vi "UHR-Fleezers Control (host) - 10.0.vi"() -> ()   [LabVIEW 2009] (continued)
  n151 = call "IMAQ Create"("Image Name"="APD 2 Image", "Image Type"=w32) -> ("New Image"=w30:T2)  [unwired: 3 in, 1 out]
  n152 = call "IMAQ Create"("Image Name"="Det. X Image", "Image Type"=w32) -> ("New Image"=w29:T2)  [unwired: 3 in, 1 out]
  n153 = call "IMAQ Create"("Image Name"="Det. Y Image", "Image Type"=w32) -> ("New Image"=w28:T2)  [unwired: 3 in, 1 out]
  n154 = call-poly "VISA Configure Serial Port"("VISA resource name"="Harvard Syringe Pump Serial Port", "baud rate (9600)"=u32 115200, "stop bits (10: 1 bit)"=w25) -> ("VISA resource name out"=w22:refnum<visa-resource-name>, "error out"=w23:errorcluster)  [unwired: 4 in, 7 out]
  n155 = Bundle("New Image"=w31, "New Image"=w30, "New Image"=w29, "New Image"=w28) -> (w27:T21)  [unwired: 1 in]
  n156 = node-c288(i64 1 ("Period")) -> (w157:T22)  [unwired: 3 out]
  n157 = node-c288() -> (w52:T22)  [unwired: 4 out]
  n158 = node-c288() -> (w50:T22)  [unwired: 4 out]
  n159 = node-c288() -> (w54:T22)  [unwired: 4 out]
  n160 = node-c288() -> (w39:T22)  [unwired: 4 in]
  n161 = timed-loop "Acquire Data" {
    tunnel: w107 -> [w951]
    tunnel: w106 -> [w950]
    tunnel: [w984] -> w254
    tunnel: [w978] -> w252
    timing: w157 -> [_]
    timing-out: [_] -> w156
    tunnel: w27 -> [w773]
    stop <- "Stop All" stop-if-true
    w757 = "NI_ChannelName" ("name")
    n162 = node-c288() -> ()  [unwired: 2 out]
    n163 = case "Reset data stream" shown="True" "Reset" {
      tunnel: w951 -> [w3448 w3460]
      tunnel: w950 -> [w3447 w3459]
      tunnel: [w3448 w3457] -> w946
      tunnel: [w3447 w3456] -> w945
      frame #0 {
      }
      frame #1 {
        w3458 = TRUE ("AI to FIFO")
        w3464 = FALSE ("AI to FIFO")
        n164 = local write "Overflow (data lost)"(FALSE ("Overflow (data lost)")) -> ()
        n165 = xnode "Read/Write Control"("FPGA VI Reference In"=w3460, "error in"=w3459, "AI to FIFO"=w3464, "APD to FIFO"=w3464) -> ("FPGA VI Reference Out"=w3452:T20, "error out"=w3463:errorcluster)
        n166 = xnode "Invoke Method"("FPGA VI Reference In"=w3451, "error in"=w3463) -> ("FPGA VI Reference Out"=w3461:T20, "error out"=w3462:errorcluster)
        n167 = xnode "Invoke Method"("FPGA VI Reference In"=w3461, "error in"=w3462) -> ("FPGA VI Reference Out"=w3455:T20, "error out"=w3454:errorcluster)
        n168 = flat-sequence {
          tunnel: w3452 -> [w3469]
          tunnel: [w3469] -> w3451
          frame #0 {
            n169 = Wait (ms)(milliseconds to wait=u32 1000) -> ()  [unwired: 1 out]
          }
        }
        n170 = xnode "Invoke Method"("FPGA VI Reference In"=w3455, "error in"=w3454) -> ("FPGA VI Reference Out"=w3450:T20, "error out"=w3453:errorcluster)
        n171 = flat-sequence {
          tunnel: w3450 -> [w3467]
          tunnel: [w3467] -> w3449
          frame #0 {
            n172 = Wait (ms)(milliseconds to wait=u32 1000) -> ()  [unwired: 1 out]
          }
        }
        n173 = xnode "Read/Write Control"("FPGA VI Reference In"=w3449, "error in"=w3453, "AI to FIFO"=w3458, "APD to FIFO"=w3458) -> ("FPGA VI Reference Out"=w3457:T20, "error out"=w3456:errorcluster)
      }
    }
    n174 = Or(x="Start AOD Scan", y="Trap Raster Scan") -> (x .or. y?=w896:bool)
    n175 = And(x="Save scans", y=w896) -> (x .and. y?=w942:bool)
    n176 = case "Start AOM raster scan" shown="True" w896 {
      tunnel: w946 -> [w2584 w2594]
      tunnel: w945 -> [w2583 w2593]
      tunnel: [w2584 w2587] -> w944
      tunnel: [w2583 w2586] -> w943
      frame #0 {
      }
      frame #1 {
        n177 = case shown="True" "Restart DMA? (AOD)" {
          tunnel: [w2960 w2962] -> w2588
          tunnel: [w2959 w2961] -> w2589
          tunnel: w2594 -> [w2960 w2970]
          tunnel: w2593 -> [w2959 w2969]
          frame #0 {
          }
          frame #1 {
            w2966 = FALSE ("AI to FIFO")
            n178 = xnode "Read/Write Control"("FPGA VI Reference In"=w2970, "error in"=w2969, "AI to FIFO"=w2966, "APD to FIFO"=w2966) -> ("FPGA VI Reference Out"=w2968:T20, "error out"=w2967:errorcluster)
            n179 = xnode "Invoke Method"("FPGA VI Reference In"=w2968, "error in"=w2967) -> ("FPGA VI Reference Out"=w2972:T20, "error out"=w2971:errorcluster)
            n180 = local write "Overflow (data lost)"(FALSE ("Overflow (data lost)")) -> ()
            n181 = xnode "Invoke Method"("FPGA VI Reference In"=w2972, "error in"=w2971) -> ("FPGA VI Reference Out"=w2964:T20, "error out"=w2963:errorcluster)
            n182 = xnode "Invoke Method"("FPGA VI Reference In"=w2964, "error in"=w2963) -> ("FPGA VI Reference Out"=w2962:T20, "error out"=w2961:errorcluster)
          }
        }
        n183 = case shown="True" "Move MCL Also?" {
          tunnel: w2589 -> [w2597 w2703]
          tunnel: w2588 -> [w2598 w2704]
          tunnel: [w2596 w2707] -> w2587
          tunnel: [w2595 w2706] -> w2586
          frame #0 {
            w2599 = TRUE ("AI to FIFO")
            n184 = xnode "Read/Write Control"("FPGA VI Reference In"=w2598, "error in"=w2597, "AI to FIFO"=w2599, "APD to FIFO"=w2599, "Start scan"=w2599) -> ("FPGA VI Reference Out"=w2596:T20, "error out"=w2595:errorcluster)
          }
          frame #1 {
            w2700 = FALSE ("1D or 2D Scan?")
            w2705 = TRUE ("AI to FIFO")
            # "Count for MCL loop"
            # "N total cycles"
            # "N steps"
            # "V_int"
            n185 = local read "Scan Range (nm)"() -> (w2682:dbl)
            n186 = local read "Number of F/B Scans (AOD)"() -> (w2699:u16)
            n187 = Sign(1:w2682) -> (0:w2681:dbl)
            n188 = Compound Arithmetic op=MULTIPLY(w2682, "MCL Step Position Ratio", "MCL/AOM Scale Tweak") -> (w2686:dbl)
            n189 = Negate(x=w2681) -> (-x=w2678:dbl)
            n190 = Multiply(x=w2678, y="MCL Step Increment (V_int)") -> (x*y=w2680:dbl)
            n191 = Divide(x=w2686, y="MCL X Cal (nm/V)") -> (x/y=w2692:dbl)
            n192 = Multiply(x=32767.0 ("y"), y=w2692) -> (x*y=w2698:dbl)
            n193 = local read "Total Counts (ticks)"() -> (w2683:u32)
            n194 = local read "Cycles/step (AOD)"() -> (w2694:u64)
            n195 = local read "Scan steps (AOD)"() -> (w2695:u64)
            n196 = Divide(x=w2698, y=10.0) -> (x/y=w2691:dbl)
            n197 = Divide(x=w2691, y="MCL Step Increment (V_int)") -> (x/y=w2689:dbl)
            n198 = Absolute Value(x=w2689) -> (abs(x)=w2677:dbl)
            n199 = Compound Arithmetic op=MULTIPLY(w2695, w2694, w2683) -> (w2690:u64)
            n200 = local write "wait to reset values"(w2705) -> ()
            n201 = local write "MCL Scanning"(w2705) -> ()
            n202 = Divide(x=w2690, y=w2677) -> (x/y=w2687:dbl)
            "MCL Count" <- w2687
            n203 = xnode "Read/Write Control"("FPGA VI Reference In"=w2704, "error in"=w2703, "Scan steps (MCL)"=w2677, "Number of scans (MCL)"=w2699, "Cycles per step (MCL)"=u64 1, "Scan freq.  increment (MCL)"=w2680, "1D or 2D Scan?"=w2700, "MCL Scan Axis"=w2700, "Cont. Scan (MCL)"=w2700, "MCL count"=w2687) -> ("FPGA VI Reference Out"=w2702:T20, "error out"=w2701:errorcluster)
            n204 = xnode "Read/Write Control"("FPGA VI Reference In"=w2702, "error in"=w2701, "AI to FIFO"=w2705, "APD to FIFO"=w2705, "Start scan"=w2705, "Start scan (MCL)"=w2705) -> ("FPGA VI Reference Out"=w2707:T20, "error out"=w2706:errorcluster)
          }
        }
        n205 = local write "Trap Raster Scan"(FALSE ("Trap Raster Scan")) -> ()
        "Raster Scanning..." <- TRUE ("Scanning...")
      }
    }
    n206 = Compound Arithmetic op=OR("Start MCL Scan", "Confocal Image", "Confocal Linescan") -> (w894:bool)
    n207 = And(x="Save Data (MCL)", y=w894) -> (x .and. y?=w941:bool)
    n208 = case "Start MCL raster scan" shown="True" w894 {
      tunnel: w944 -> [w1743 w1758]
      tunnel: w943 -> [w1742 w1757]
      tunnel: [w1743 w1753] -> w771
      tunnel: [w1742 w1752] -> w770
      tunnel: [FALSE w1751] -> w927
      tunnel: "Start MCL Scan" -> [_ w1746]
      tunnel: "Confocal Image" -> [_ w1745]
      tunnel: "Confocal Linescan" -> [_ _]
      frame #0 {
      }
      frame #1 {
        w1751 = TRUE
        n209 = case shown="True" "Restart DMA? (MCL)" {
          tunnel: [w1995 w1997] -> w1756
          tunnel: [w1994 w1996] -> w1755
          tunnel: w1758 -> [w1995 w2005]
          tunnel: w1757 -> [w1994 w2004]
          frame #0 {
          }
          frame #1 {
            w2001 = FALSE ("AI to FIFO")
            n210 = xnode "Read/Write Control"("FPGA VI Reference In"=w2005, "error in"=w2004, "AI to FIFO"=w2001, "APD to FIFO"=w2001) -> ("FPGA VI Reference Out"=w2003:T20, "error out"=w2002:errorcluster)
            n211 = xnode "Invoke Method"("FPGA VI Reference In"=w2003, "error in"=w2002) -> ("FPGA VI Reference Out"=w2007:T20, "error out"=w2006:errorcluster)
            n212 = xnode "Invoke Method"("FPGA VI Reference In"=w2007, "error in"=w2006) -> ("FPGA VI Reference Out"=w1999:T20, "error out"=w1998:errorcluster)
            n213 = xnode "Invoke Method"("FPGA VI Reference In"=w1999, "error in"=w1998) -> ("FPGA VI Reference Out"=w1997:T20, "error out"=w1996:errorcluster)
            n214 = local write "Overflow (data lost)"(FALSE ("Overflow (data lost)")) -> ()
          }
        }
        n215 = case shown="False" w1746 {
          selector: w1746 -> [_ w1762]
          tunnel: w1745 -> [w1761 _]
          tunnel: [w1761 w1762] -> w1744
          frame #0 {
            n216 = property on="2D or 1D Scan" class="Bool (strict)"("Val(Sgnl)"=w1761) -> ()  [unwired: 2 in, 2 out]
            n217 = property on="Confocal Image" class="Bool (strict)"("Value"=FALSE ("Start Confocal Map")) -> ()  [unwired: 2 in, 2 out]
          }
          frame #1 {
          }
        }
        n218 = local write "MCL Scanning"(w1751) -> ()
        n219 = local read "AO1"() -> (w1748:dbl)
        n220 = local read "AO2"() -> (w1747:dbl)
        n221 = case shown="True" "Center Scan" {
          tunnel: w1756 -> [w1769 w1878]
          tunnel: w1755 -> [w1768 w1877]
          tunnel: [w1767 w1876] -> w1753
          tunnel: [w1766 w1875] -> w1752
          tunnel: [w1764 w1862] -> w1750
          tunnel: [w1763 w1861] -> w1749
          tunnel: w1748 -> [w1764 w1867]
          tunnel: w1747 -> [w1763 w1870]
          tunnel: w1744 -> [_ _]
          frame #0 {
            w1765 = TRUE ("AI to FIFO")
            n222 = xnode "Read/Write Control"("FPGA VI Reference In"=w1769, "error in"=w1768, "AI to FIFO"=w1765, "APD to FIFO"=w1765, "Start scan (MCL)"=w1765) -> ("FPGA VI Reference Out"=w1767:T20, "error out"=w1766:errorcluster)
          }
          frame #1 {
            w1874 = TRUE ("AI to FIFO")
            n223 = local read "Scan steps (MCL)"() -> (w1853:u64)
            n224 = local read "Scan lines (y)"() -> (w1849:u64)
            n225 = local read "Fast Scan Dir"() -> (w1860:bool)
            n226 = local read "Actual MCL Inc (V)"() -> (w1850:dbl)
            n227 = Decrement(x=w1849) -> (x-1=w1848:u64)
            n228 = Decrement(x=w1853) -> (x-1=w1852:u64)
            n229 = Multiply(x=w1850, y=w1848) -> (x*y=w1847:dbl)
            n230 = Divide(x=w1847, y=2.0) -> (x/y=w1857:dbl)
            n231 = Multiply(x=w1850, y=w1852) -> (x*y=w1851:dbl)
            n232 = Divide(x=w1851, y=2.0) -> (x/y=w1856:dbl)
            n233 = Select(t=w1856, s=w1860, f=w1857) -> (s? t:f=w1855:dbl)
            n234 = Select(t=w1857, s=w1860, f=w1856) -> (s? t:f=w1859:dbl)
            n235 = Subtract(x=w1867, y=w1859) -> (x-y=w1858:dbl)
            n236 = Subtract(x=w1870, y=w1855) -> (x-y=w1854:dbl)
            n237 = local read "2D or 1D Scan"() -> (w1872:bool)
            n238 = Not(x=w1860) -> (.not. x?=w1866:bool)
            n239 = Not(x=w1872) -> (.not. x?=w1868:bool)
            n240 = And(x=w1860, y=w1868) -> (x .and. y?=w1869:bool)
            n241 = And(x=w1868, y=w1866) -> (x .and. y?=w1871:bool)
            n242 = Select(t=w1870, s=w1871, f=w1854) -> (s? t:f=w1861:dbl)
            n243 = Select(t=w1867, s=w1869, f=w1858) -> (s? t:f=w1862:dbl)
            n244 = call "Volt to I16.vi"("Voltage In"=w1862) -> ("I16 Voltage Out"=w1865:i16)
            n245 = call "Volt to I16.vi"("Voltage In"=w1861) -> ("I16 Voltage Out"=w1864:i16)
            n246 = xnode "Read/Write Control"("FPGA VI Reference In"=w1878, "error in"=w1877, "AI to FIFO"=w1874, "APD to FIFO"=w1874, "Start scan (MCL)"=w1874, "AO1"=w1865, "AO2"=w1864) -> ("FPGA VI Reference Out"=w1876:T20, "error out"=w1875:errorcluster)
          }
        }
        "Initial Y" <- w1750
        "Initial X" <- w1749
        "wait to reset values" <- w1751
      }
    }
    n247 = local read "Trap Pos Elements/DMA read"() -> (w767:u32)
    n248 = local read "Trap AI Elements/DMA read"() -> (w855:u32)
    n249 = local read "APD Elements/DMA read"() -> (w812:u32)
    n250 = xnode "Get APD Data"("FPGA VI Reference In"=w771, "error in"=w770, "Number of Elements"=w812, "Timeout (ms)"=-1) -> ("Data"=w811:u32[], "Elements Remaining"=→"APD FIFO Elements Remaining":u32)  [unwired: 2 out]
    n251 = xnode "Invoke Method"("FPGA VI Reference In"=w771, "error in"=w770, "Number of Elements"=w767, "Timeout (ms)"=-1) -> ("Data"=w766:u64[], "Elements Remaining"=→"Trap Pos FIFO El Remaining":u32)  [unwired: 2 out]
    n252 = xnode "Get Trap Data"("FPGA VI Reference In"=w771, "error in"=w770, "Number of Elements"=w855, "Timeout (ms)"=-1 ("Timeout")) -> ("FPGA VI Reference Out"=w842:T20, "error out"=w841:errorcluster, "Data"=w964:u32[], "Elements Remaining"=w993:u32)
    "FIFO El. Rem." <- w993
    n253 = local read "Trap AI FIFO Depth"() -> (w995:u32)
    n254 = call "IR AOM word to freq - vec.vi"("Frequency Word In (double vec)"=w766) -> ("Frequency Out"=w765:dbl[])
    n255 = Subtract(x=w995, y=w855) -> (x-y=w994:u32)
    n256 = Divide(x=w993, y=w994) -> (x/y=w992:dbl)
    "Buffer Status" <- w992
    n257 = Decimate 1D Array(w765) -> (w764:dbl[], w763:dbl[])
    n258 = Equal?(x=w992, y=1.0) -> (x = y?=w990:bool)
    n259 = Build Array(w764, w763) -> (w762:dbl[][])
    n260 = case "Alert buffer overflow" shown="True" w990 {
      frame #0 {
      }
      frame #1 {
        n261 = call <vilib>:"Beep.vi"() -> ()  [unwired: 3 in, 9 out]
        "Overflow (data lost)" <- TRUE ("Overflow (data lost)")
      }
    }
    n262 = local read "FPGA Averaging"() -> (w854:bool)
    n263 = case "Special unpacking case if no averaging done by FPGA" shown="False" w854 {
      tunnel: w964 -> [w2181 w2207]
      tunnel: [w2152 w2182] -> w963
      frame #0 {
        n264 = Decimate 1D Array(w2181) -> (w2180:u32[], w2179:u32[], w2178:u32[], w2177:u32[])
        n265 = Split Number(x=w2180) -> (hi(x)=w2176:u16[], lo(x)=w2175:u16[])
        n266 = Split Number(x=w2179) -> (hi(x)=w2174:u16[], lo(x)=w2173:u16[])
        n267 = Split Number(x=w2178) -> (hi(x)=w2172:u16[], lo(x)=w2171:u16[])
        n268 = Split Number(x=w2177) -> (hi(x)=w2170:u16[], lo(x)=w2169:u16[])
        n269 = To Word Integer(number=w2176) -> (16bit integer=w2168:i16[])
        n270 = To Word Integer(number=w2175) -> (16bit integer=w2167:i16[])
        n271 = To Word Integer(number=w2174) -> (16bit integer=w2166:i16[])
        n272 = To Word Integer(number=w2173) -> (16bit integer=w2165:i16[])
        n273 = To Word Integer(number=w2172) -> (16bit integer=w2164:i16[])
        n274 = To Word Integer(number=w2171) -> (16bit integer=w2163:i16[])
        n275 = To Word Integer(number=w2170) -> (16bit integer=w2162:i16[])
        n276 = To Word Integer(number=w2169) -> (16bit integer=w2161:i16[])
        n277 = To Double Precision Float(number=w2168) -> (double precision float=w2160:dbl[])
        n278 = To Double Precision Float(number=w2167) -> (double precision float=w2159:dbl[])
        n279 = To Double Precision Float(number=w2166) -> (double precision float=w2158:dbl[])
        n280 = To Double Precision Float(number=w2165) -> (double precision float=w2157:dbl[])
        n281 = To Double Precision Float(number=w2164) -> (double precision float=w2156:dbl[])
        n282 = To Double Precision Float(number=w2163) -> (double precision float=w2155:dbl[])
        n283 = To Double Precision Float(number=w2162) -> (double precision float=w2154:dbl[])
        n284 = To Double Precision Float(number=w2161) -> (double precision float=w2153:dbl[])
        n285 = Interleave 1D Arrays(w2160, w2159, w2158, w2157, w2156, w2155, w2154, w2153) -> (w2152:dbl[])
      }
      frame #1 {
        n286 = Decimate 1D Array(w2207) -> (w2198:u32[], w2196:u32[], w2194:u32[], w2192:u32[], w2190:u32[], w2188:u32[], w2186:u32[], w2184:u32[])
        n287 = To Long Integer(number=w2198) -> (32bit integer=w2206:i32[])
        n288 = To Long Integer(number=w2196) -> (32bit integer=w2205:i32[])
        n289 = To Long Integer(number=w2194) -> (32bit integer=w2204:i32[])
        n290 = To Long Integer(number=w2192) -> (32bit integer=w2203:i32[])
        n291 = To Long Integer(number=w2190) -> (32bit integer=w2202:i32[])
        n292 = To Long Integer(number=w2188) -> (32bit integer=w2201:i32[])
        n293 = To Long Integer(number=w2186) -> (32bit integer=w2200:i32[])
        n294 = To Long Integer(number=w2184) -> (32bit integer=w2199:i32[])
        n295 = To Double Precision Float(number=w2206) -> (double precision float=w2197:dbl[])
        n296 = To Double Precision Float(number=w2205) -> (double precision float=w2195:dbl[])
        n297 = To Double Precision Float(number=w2204) -> (double precision float=w2193:dbl[])
        n298 = To Double Precision Float(number=w2203) -> (double precision float=w2191:dbl[])
        n299 = To Double Precision Float(number=w2202) -> (double precision float=w2189:dbl[])
        n300 = To Double Precision Float(number=w2201) -> (double precision float=w2187:dbl[])
        n301 = To Double Precision Float(number=w2200) -> (double precision float=w2185:dbl[])
        n302 = To Double Precision Float(number=w2199) -> (double precision float=w2183:dbl[])
        n303 = Interleave 1D Arrays(w2197, w2195, w2193, w2191, w2189, w2187, w2185, w2183) -> (w2182:dbl[])
      }
    }
    n304 = local read "FPGA Ave."() -> (w853:dbl)
    n305 = local read "Trap Sets"() -> (w852:i16)
    n306 = Divide(x=w963, y=w853) -> (x/y=w970:dbl[])
    n307 = case "Deinterlace trap data, average down PSD" shown="2" w852 {
      tunnel: w970 -> [w2225 w2290]
      tunnel: [w2222 w2287] -> w845
      tunnel: [w2225 w2289] -> w744
      tunnel: "Detector Type" -> [w2224 w2285]
      tunnel: [w2223 w2288] -> w844
      tunnel: [w2221 w2286] -> w962
      frame #0 {
        n308 = Divide(x=w2225, y=3276.7) -> (x/y=w2226:dbl[])
        n309 = Decimate 1D Array(w2226) -> (w2235:dbl[], w2234:dbl[], w2233:dbl[], w2232:dbl[], w2231:dbl[], w2230:dbl[], w2229:dbl[], w2228:dbl[])
        n310 = case shown="\"IR-QPD + PSD + FB-QPD position\"" w2224 {
          tunnel: w2235 -> [w2259 w2284]
          tunnel: w2234 -> [w2258 w2283]
          tunnel: w2233 -> [w2243 w2261]
          tunnel: w2232 -> [w2244 w2271]
          tunnel: w2231 -> [w2257 w2282]
          tunnel: w2230 -> [w2256 w2281]
          tunnel: w2229 -> [w2240 w2262]
          tunnel: w2228 -> [w2239 w2260]
          tunnel: [w2238 w2268] -> w2223
          tunnel: [w2237 w2267] -> w2222
          tunnel: [w2236 w2266] -> w2221
          frame #0 {
            w2236 = 0  # Channel pattern
            n311 = Divide(x=w2259, y=w2244) -> (x/y=w2246:dbl[])
            n312 = Divide(x=w2258, y=w2244) -> (x/y=w2245:dbl[])
            n313 = Divide(x=w2257, y=w2240) -> (x/y=w2242:dbl[])
            n314 = Divide(x=w2256, y=w2239) -> (x/y=w2241:dbl[])
            n315 = Build Array(w2246, w2245, w2244, w2243, w2242, w2241, w2240, w2239) -> (w2237:dbl[][])
            n316 = Bundle("T1 Y", "T1 X", "T1 Sum", "FB Sum", "PSD Y", "PSD X", "PSD Y Sum", "PSD X Sum") -> (w2255:T34)  [unwired: 1 out]
            n317 = Cluster To Array(cluster=w2255) -> (array=w2238:string[])
          }
          frame #1 {
            w2266 = 3  # Channel pattern
            n318 = Negate(x=w2262) -> (-x=w2263:dbl[])
            n319 = Divide(x=w2284, y=w2271) -> (x/y=w2273:dbl[])
            n320 = Divide(x=w2283, y=w2271) -> (x/y=w2272:dbl[])
            n321 = Divide(x=w2282, y=w2262) -> (x/y=w2270:dbl[])
            n322 = Divide(x=w2281, y=w2263) -> (x/y=w2269:dbl[])
            n323 = Build Array(w2273, w2272, w2271, w2260, w2261, w2270, w2269, w2262) -> (w2267:dbl[][])
            n324 = Bundle("T1 Y", "T1 X", "T1 Sum", "FB X", "FB Sum", "PSD Y", "PSD X", "PSD Y Sum") -> (w2280:T34)  [unwired: 1 out]
            n325 = Cluster To Array(cluster=w2280) -> (array=w2268:string[])
          }
        }
      }
      frame #1 {
        n326 = case shown="\"IR-QPD + PSD + FB-QPD X position\"" w2285 {
          tunnel: w2290 -> [w2351 w2418 w2488]
          tunnel: [w2331 w2403 w2475] -> w2289
          tunnel: [w2317 w2394 w2466] -> w2288
          tunnel: [w2316 w2354 w2433] -> w2287
          tunnel: [w2310 w2392 w2464] -> w2286
          frame #0 {
            w2310 = 1  # Channel pattern
            # "time average x2 the 4th signal and the 4 psd signals (detection laser)"
            # "deinterlace 3 signals from qpd"
            n327 = Decimate 1D Array(w2351) -> (w2350:dbl[], w2349:dbl[], w2315:dbl[], w2348:dbl[], w2338:dbl[], w2336:dbl[], w2335:dbl[], w2333:dbl[])
            n328 = Decimate 1D Array(w2315) -> (w2314:dbl[], w2313:dbl[])
            n329 = Decimate 1D Array(w2350) -> (w2347:dbl[], w2319:dbl[])
            n330 = Decimate 1D Array(w2349) -> (w2346:dbl[], w2344:dbl[])
            n331 = Decimate 1D Array(w2348) -> (w2345:dbl[], w2343:dbl[])
            n332 = call "downsample 1D array - double.vi"("Ave N"=2.0, "Array In"=w2338) -> ("Array Out"=w2337:dbl[])  [unwired: 1 out]
            n333 = call "downsample 1D array - double.vi"("Ave N"=2.0, "Array In"=w2336) -> ("Array Out"=w2318:dbl[])  [unwired: 1 out]
            n334 = call "downsample 1D array - double.vi"("Ave N"=2.0, "Array In"=w2335) -> ("Array Out"=w2334:dbl[])  [unwired: 1 out]
            n335 = call "downsample 1D array - double.vi"("Ave N"=2.0, "Array In"=w2333) -> ("Array Out"=w2332:dbl[])  [unwired: 1 out]
            n336 = Interleave 1D Arrays(w2347, w2346, w2345, w2319, w2344, w2343, w2314, w2313, w2337, w2318, w2334, w2332) -> (w2331:dbl[])
            n337 = Divide(x=w2331, y=3276.7) -> (x/y=w2330:dbl[])
            n338 = Decimate 1D Array(w2330) -> (w2329:dbl[], w2328:dbl[], w2327:dbl[], w2326:dbl[], w2325:dbl[], w2324:dbl[], w2312:dbl[], w2311:dbl[], w2323:dbl[], w2322:dbl[], w2321:dbl[], w2320:dbl[])
            n339 = Divide(x=w2329, y=w2327) -> (x/y=w2297:dbl[])
            n340 = Divide(x=w2328, y=w2327) -> (x/y=w2296:dbl[])
            n341 = Divide(x=w2326, y=w2324) -> (x/y=w2295:dbl[])
            n342 = Divide(x=w2325, y=w2324) -> (x/y=w2294:dbl[])
            n343 = Divide(x=w2323, y=w2321) -> (x/y=w2293:dbl[])
            n344 = Divide(x=w2322, y=w2320) -> (x/y=w2292:dbl[])
            n345 = Build Array(w2297, w2296, w2327, w2295, w2294, w2324, w2312, w2311, w2293, w2292, w2321, w2320) -> (w2316:dbl[][])
            n346 = Bundle("T1 Y", "T1 X", "T1 Sum", "T2 Y", "T2 X", "T2 Sum", "T1 FB Sum", "T2 FB Sum", "PSD Y", "PSD X", "PSD Y Sum", "PSD X Sum") -> (w2298:T35)  [unwired: 1 out]
            n347 = Cluster To Array(cluster=w2298) -> (array=w2317:string[])
          }
          frame #1 {
            w2392 = 2  # Channel pattern
            # "time average x2 the 3 psd signals (detection laser)"
            # "deinterlace 3 signals from qpds"
            n348 = Decimate 1D Array(w2418) -> (w2417:dbl[], w2416:dbl[], w2393:dbl[], w2415:dbl[], w2406:dbl[], w2405:dbl[], w2404:dbl[], w2380:dbl[])
            n349 = Decimate 1D Array(w2393) -> (w2375:dbl[], w2373:dbl[])
            n350 = Decimate 1D Array(w2417) -> (w2414:dbl[], w2395:dbl[])
            n351 = Decimate 1D Array(w2416) -> (w2413:dbl[], w2411:dbl[])
            n352 = Decimate 1D Array(w2415) -> (w2412:dbl[], w2410:dbl[])
            n353 = Decimate 1D Array(w2380) -> (w2376:dbl[], w2374:dbl[])
            n354 = call "downsample 1D array - double.vi"("Ave N"=2.0, "Array In"=w2406) -> ("Array Out"=w2379:dbl[])  [unwired: 1 out]
            n355 = call "downsample 1D array - double.vi"("Ave N"=2.0, "Array In"=w2405) -> ("Array Out"=w2378:dbl[])  [unwired: 1 out]
            n356 = call "downsample 1D array - double.vi"("Ave N"=2.0, "Array In"=w2404) -> ("Array Out"=w2377:dbl[])  [unwired: 1 out]
            n357 = Interleave 1D Arrays(w2414, w2413, w2412, w2395, w2411, w2410, w2376, w2375, w2374, w2373, w2379, w2378, w2377) -> (w2403:dbl[])
            n358 = Divide(x=w2403, y=3276.7) -> (x/y=w2402:dbl[])
            n359 = Decimate 1D Array(w2402) -> (w2401:dbl[], w2400:dbl[], w2399:dbl[], w2398:dbl[], w2397:dbl[], w2396:dbl[], w2365:dbl[], w2363:dbl[], w2362:dbl[], w2360:dbl[], w2359:dbl[], w2358:dbl[], w2355:dbl[])
            n360 = Negate(x=w2355) -> (-x=w2353:dbl[])
            n361 = Divide(x=w2359, y=w2355) -> (x/y=w2357:dbl[])
            n362 = Divide(x=w2358, y=w2353) -> (x/y=w2356:dbl[])
            n363 = Divide(x=w2401, y=w2399) -> (x/y=w2384:dbl[])
            n364 = Divide(x=w2400, y=w2399) -> (x/y=w2383:dbl[])
            n365 = Divide(x=w2398, y=w2396) -> (x/y=w2382:dbl[])
            n366 = Divide(x=w2397, y=w2396) -> (x/y=w2381:dbl[])
            n367 = Divide(x=w2365, y=w2363) -> (x/y=w2364:dbl[])
            n368 = Divide(x=w2362, y=w2360) -> (x/y=w2361:dbl[])
            n369 = Build Array(w2384, w2383, w2399, w2382, w2381, w2396, w2364, w2363, w2361, w2360, w2357, w2356, w2355) -> (w2354:dbl[][])
            n370 = Bundle("T1 Y", "T1 X", "T1 Sum", "T2 Y", "T2 X", "T2 Sum", "T1 FB X", "T1 FB Sum", "T2 FB X", "T2 FB Sum", "PSD Y", "PSD X", "PSD Y Sum") -> (w2385:T36)  [unwired: 1 out]
            n371 = Cluster To Array(cluster=w2385) -> (array=w2394:string[])
          }
          frame #2 {
            w2464 = 4  # Channel pattern
            # "time average x2 the 3 psd signals (detection laser)"
            # "deinterlace 3 signals from qpds"
            n372 = Decimate 1D Array(w2488) -> (w2487:dbl[], w2486:dbl[], w2465:dbl[], w2485:dbl[], w2431:dbl[], w2477:dbl[], w2476:dbl[], w2453:dbl[])
            n373 = Decimate 1D Array "Feedback Sum"(w2465) -> (w2449:dbl[], w2447:dbl[])
            n374 = Decimate 1D Array "QPD Y"(w2487) -> (w2484:dbl[], w2467:dbl[])
            n375 = Decimate 1D Array "QPD X"(w2486) -> (w2483:dbl[], w2481:dbl[])
            n376 = Decimate 1D Array "Feedback Y"(w2431) -> (w2430:dbl[], w2429:dbl[])
            n377 = Decimate 1D Array "QPD Sum"(w2485) -> (w2482:dbl[], w2480:dbl[])
            n378 = Decimate 1D Array "Feedback X"(w2453) -> (w2450:dbl[], w2448:dbl[])
            n379 = call "downsample 1D array - double.vi"("Ave N"=2.0, "Array In"=w2477) -> ("Array Out"=w2452:dbl[])  [unwired: 1 out]
            n380 = call "downsample 1D array - double.vi"("Ave N"=2.0, "Array In"=w2476) -> ("Array Out"=w2451:dbl[])  [unwired: 1 out]
            n381 = Interleave 1D Arrays(w2484, w2483, w2482, w2467, w2481, w2480, w2430, w2450, w2449, w2429, w2448, w2447, w2452, w2451) -> (w2475:dbl[])
            n382 = Divide(x=w2475, y=3276.7) -> (x/y=w2474:dbl[])
            n383 = Decimate 1D Array(w2474) -> (w2473:dbl[], w2472:dbl[], w2471:dbl[], w2470:dbl[], w2469:dbl[], w2468:dbl[], w2426:dbl[], w2440:dbl[], w2424:dbl[], w2425:dbl[], w2438:dbl[], w2422:dbl[], w2436:dbl[], w2434:dbl[])
            n384 = Negate(x=w2434) -> (-x=w2432:dbl[])
            n385 = Divide(x=w2436, y=w2432) -> (x/y=w2435:dbl[])
            n386 = Divide(x=w2425, y=w2422) -> (x/y=w2421:dbl[])
            n387 = Divide(x=w2426, y=w2424) -> (x/y=w2423:dbl[])
            n388 = Divide(x=w2473, y=w2471) -> (x/y=w2457:dbl[])
            n389 = Divide(x=w2472, y=w2471) -> (x/y=w2456:dbl[])
            n390 = Divide(x=w2470, y=w2468) -> (x/y=w2455:dbl[])
            n391 = Divide(x=w2469, y=w2468) -> (x/y=w2454:dbl[])
            n392 = Divide(x=w2440, y=w2424) -> (x/y=w2439:dbl[])
            n393 = Divide(x=w2438, y=w2422) -> (x/y=w2437:dbl[])
            n394 = Build Array(w2457, w2456, w2471, w2455, w2454, w2468, w2423, w2439, w2424, w2421, w2437, w2422, w2435, w2434) -> (w2433:dbl[][])
            n395 = Bundle("T1 Y", "T1 X", "T1 Sum", "T2 Y", "T2 X", "T2 Sum", "T1 FB Y", "T1 FB X", "T1 FB Sum", "T2 FB Y", "T2 FB X", "T2 FB Sum", "PSD X", "PSD Y Sum") -> (w2420:T37)  [unwired: 1 out]
            n396 = Cluster To Array(cluster=w2420) -> (array=w2466:string[])
          }
        }
      }
    }
    "AI labels" <- w844
    n397 = To Word Integer(number=w744) -> (16bit integer=w749:i16[])
    n398 = Decimate 1D Array(w811) -> (w840:u32[], w775:u32[])
    n399 = local read "DMA Update Period (s)"() -> (w856:dbl)
    n400 = Build Array(w840, w775) -> (w924:u32[][])
    n401 = local read "Data Period (s)"() -> (w825:dbl)
    n402 = Decimate 1D Array(w744) -> (w742:dbl[], w741:dbl[], w739:dbl[], w738:dbl[])  [unwired: 9 out]
    n403 = To Double Precision Float(number=w924) -> (double precision float=w925:dbl[][])
    n404 = local read "APD Integration Time (s)"() -> (w788:dbl)
    n405 = Divide(x=w742, y=w741) -> (x/y=w743:dbl[])
    n406 = Divide(x=w739, y=w738) -> (x/y=w740:dbl[])
    n407 = feedback #1(0.0) -> (w759:dbl)
    n408 = Add(x=w856, y=w759) -> (x+y=w966:dbl)
    n409 = To Time Stamp(1:w759) -> (0:w758:timestamp)
    n410 = Split 1D Array(array=w743, index="N El. to Ave.") -> (second subarray=w747:dbl[])  [unwired: 1 out]
    n411 = Split 1D Array(array=w740, index="N El. to Ave.") -> (second subarray=w746:dbl[])  [unwired: 1 out]
    n412 = local read "Trap X AI1 (DMA)"() -> (w745:T10)
    n413 = Multiply(x=w825, y="Trap Disp. Downsample") -> (x*y=w760:dbl)
    "Display Period (s)" <- w760
    n414 = for "Trap AI" {
      tunnel: [w2220] -> w958 mode=indexing
      tunnel: w758 -> [w2210]
      tunnel: "Trap Disp. Downsample" -> [w2218]
      tunnel: w845 -> [w2216] mode=indexing
      tunnel: w825 -> [w2215]
      tunnel: w844 -> [w2214] mode=indexing
      tunnel: w757 -> [w2213]
      tunnel: [w2212] -> w799 mode=indexing
      tunnel: w760 -> [w2211]
      workers-P: _ -> [_]
      n415 = Bundle By Name("Y"=w2216, "dt"=w2215) -> (w2217:waveform(dbl))  [unwired: 1 out]
      n416 = Set Waveform Attribute(5:w2214, 6:w2213, 7:w2217) -> (3:w2212:waveform(dbl))  [unwired: 1 in, 2 out]
      n417 = call "downsample 1D array - double.vi"("Ave N"=w2218, "Array In"=w2216) -> ("Array Out"=w2219:dbl[])  [unwired: 1 out]
      n418 = Bundle By Name(cluster=w2212, "t0"=w2210, "Y"=w2219, "dt"=w2211) -> (w2220:waveform(dbl))
    }
    n419 = call <vilib>:"Mean.vi"("X"=w746) -> ("mean"=w733:dbl)  [unwired: 1 out]
    n420 = call <vilib>:"Mean.vi"("X"=w747) -> ("mean"=w734:dbl)  [unwired: 1 out]
    n421 = Reciprocal(x=w760) -> (1/x=→"Trap Disp. Freq. (Hz)":dbl)
    n422 = local read "Data points/scans (MCL)"() -> (w936:dbl)
    n423 = To Fixed-Point(number=w733) -> (fixed-point=w731:fxp<+/-,16,1>)  [unwired: 1 in]
    n424 = To Fixed-Point(number=w734) -> (fixed-point=w732:fxp<+/-,16,1>)  [unwired: 1 in]
    n425 = Bundle("Trap 1 Pos.", "Trap 2 Pos.") -> (w756:cluster{string, string})  [unwired: 1 out]
    n426 = Bundle By Name(cluster=w745, "Set 1"=w732, "Set 2"=w731) -> (→"Trap X AI1 (DMA)":T10)
    n427 = Cluster To Array(cluster=w756) -> (array=w753:string[])
    n428 = for "Trap Position" {
      tunnel: w762 -> [w1007] mode=indexing
      tunnel: "Trap Disp. Downsample" -> [w1006]
      tunnel: w760 -> [w1004]
      tunnel: w758 -> [w1003]
      tunnel: w757 -> [w1001]
      tunnel: w753 -> [w1000] mode=indexing
      tunnel: [w999] -> w752 mode=indexing
      n429 = call "downsample 1D array - double.vi"("Ave N"=w1006, "Array In"=w1007) -> ("Array Out"=w1005:dbl[])  [unwired: 1 out]
      n430 = Bundle By Name("Y"=w1005, "dt"=w1004, "t0"=w1003) -> (w1002:waveform(dbl))  [unwired: 1 out]
      n431 = Set Waveform Attribute(5:w1000, 6:w1001, 7:w1002) -> (3:w999:waveform(dbl))  [unwired: 1 in, 2 out]
    }
    "Trap Positions" <- w752
    n432 = Bundle("APD 1", "APD 2") -> (w957:cluster{string, string})  [unwired: 1 out]
    n433 = Cluster To Array(cluster=w957) -> (array=w954:string[])
    n434 = for "APD" {
      tunnel: w925 -> [w2143] mode=indexing
      tunnel: w788 -> [w2151]
      tunnel: [w2147] -> w795 mode=indexing
      tunnel: "APD Disp. Scale" -> [w2148]
      tunnel: w757 -> [w2146]
      tunnel: w954 -> [w2145] mode=indexing
      tunnel: "APD Disp. Downsample" -> [w2141]
      tunnel: [w2144] -> w953
      workers-P: _ -> [_]
      tunnel: w758 -> [w2140]
      n435 = call "integrate 1D array interval - double.vi"("Ave N"=w2141, "Array In"=w2143) -> ("Array Out"=w2142:dbl[])  [unwired: 1 out]
      n436 = Multiply(x=w2151, y=w2141) -> (x*y=w2144:dbl)
      n437 = Divide(x=w2142, y=w2148) -> (x/y=w2149:dbl[])
      n438 = Bundle By Name("t0"=w2140, "Y"=w2149, "dt"=w2144) -> (w2150:waveform(dbl))  [unwired: 1 out]
      n439 = Set Waveform Attribute(5:w2145, 6:w2146, 7:w2150) -> (3:w2147:waveform(dbl))  [unwired: 1 in, 2 out]
    }
    "APD Display Period (s)" <- w953
    n440 = Reciprocal(x=w953) -> (1/x=→"APD Display Freq. (Hz)":dbl)
    n441 = Increment(x=w936) -> (x+1=w937:dbl)
    n442 = To Double Precision Float(number=w840) -> (double precision float=w839:dbl[])
    n443 = feedback #2(w937) -> (w940:dbl)
    n444 = Select(t=0, s=w927, f=w940) -> (s? t:f=w933:dbl)
    n445 = Array Size(array=w839) -> (size(s)=w939:i32)
    n446 = Add(x=w939, y=w933) -> (x+y=w934:dbl)
    n447 = feedback #3(w840) -> (w923:u32[])
    n448 = Build Array (concatenate)(w923, w840) -> (w920:u32[])
    n449 = feedback #4(w775) -> (w794:u32[])
    n450 = Build Array (concatenate)(w794, w775) -> (w793:u32[])
    n451 = Greater?(x=w934, y=w936) -> (0:w935:bool)
    n452 = Select(t=w933, s=w935, f=w934) -> (s? t:f=w932:dbl)
    n453 = Array Size(array=w920) -> (size(s)=w917:i32)
    n454 = Array Size(array=w840) -> (size(s)=w919:i32)
    n455 = local read "MCL Scanning"() -> (w930:bool)
    n456 = local read "APD Integration Time (s)"() -> (w802:dbl)
    n457 = Build Array (concatenate)(w795, w958) -> (w797:waveform(dbl)[])
    "All Signals" <- w797
    n458 = Multiply(x=w919, y="APD Ave N") -> (x*y=w918:dbl)
    n459 = Greater?(x=w917, y=w918) -> (0:w921:bool)
    n460 = Not(x=w935) -> (.not. x?=w929:bool)
    n461 = To Double Precision Float(number=w775) -> (double precision float=w774:dbl[])
    n462 = And(x=w929, y=w930) -> (x .and. y?=w931:bool)
    n463 = case shown="True" w921 {
      tunnel: w920 -> [w1593 w1600]
      tunnel: [w1593 w1598] -> w861
      tunnel: w918 -> [_ w1595]
      tunnel: w917 -> [_ w1599]
      tunnel: w793 -> [w1592 w1597]
      tunnel: [w1592 w1594] -> w790
      frame #0 {
      }
      frame #1 {
        n464 = Subtract(x=w1599, y=w1595) -> (x-y=w1596:dbl)
        n465 = Array Subset(array=w1600, index=w1596, length=w1595) -> (w1598:u32[])
        n466 = Array Subset(array=w1597, index=w1596, length=w1595) -> (w1594:u32[])
      }
    }
    n467 = Or(x=w931, y=w927) -> (x .or. y?=w928:bool)
    n468 = Equal?(x="Tab Control 6", y=T25."High Res Display") -> (x = y?=w848:bool)
    n469 = Multiply(x="APD Disp. Scale", y=w795) -> (x*y=w804:waveform(dbl)[])
    n470 = Multiply(x="APD Disp. Downsample", y=w802) -> (x*y=w800:dbl)
    n471 = Divide(x=w804, y=w800) -> (x/y=w772:waveform(dbl)[])
    n472 = Index Array(array=w772, index=0) -> (element=w782:waveform(dbl))
    n473 = case "For computing FFTs for display" shown="True" "Compute FFT" {
      tunnel: w799 -> [_ w3132]
      frame #0 {
      }
      frame #1 {
        n474 = Build Array("FFT 1 Choice 1", "FFT 1 Choice 2", "FFT 2 Choice 1", "FFT 2 Choice 2") -> (w3125:u16[])
        n475 = Array Size(array=w3132) -> (size(s)=w3131:i32)
        n476 = feedback #5(u16[] [100, 100, 100, 100]) -> (w3126:u16[])
        n477 = feedback #6("# Spectra to Ave.") -> (w3123:dbl)
        n478 = Not Equal?(x="# Spectra to Ave.", y=w3123) -> (x != y?=w3122:bool)
        n479 = Not Equal?(x=w3125, y=w3126) -> (x != y?=w3124:bool)
        n480 = feedback #7(1.0) -> (w3109:dbl)
        n481 = Compound Arithmetic op=OR("Reset FFT", w3124, w3122) -> (w3107:bool)
        n482 = Select(t=1.0, s=w3107, f=w3109) -> (s? t:f=w3111:dbl)
        n483 = Greater?(x=w3111, y="# Spectra to Ave.") -> (0:w3130:bool)
        n484 = Increment(x=w3111) -> (x+1=w3110:dbl)
        n485 = local read "DMA Update Period (s)"() -> (w3105:dbl)
        n486 = Multiply(x="# Spectra to Ave.", y=w3105) -> (x*y=→"Ave. Time (s)":dbl)
        n487 = Build Array(cluster{"f0":dbl, "df":dbl, "magnitude":dbl[]} {"f0"=0.0, "df"=0.0, "magnitude"=[]} ("PSD")) -> (w3114:cluster{"f0":dbl, "df":dbl, "magnitude":dbl[]}[])
        n488 = Build Array(w3114, w3114, w3114, w3114) -> (w3116:T38)
        n489 = feedback #8(w3116) -> (w3121:T38)
        n490 = for {
          N: 4 -> [_]
          tunnel: w3125 -> [w3154] mode=indexing
          tunnel: w3132 -> [w3155]
          tunnel: w3131 -> [w3157]
          tunnel: w3107 -> [w3150]
          tunnel: w3130 -> [w3149]
          tunnel: "# Spectra to Ave." -> [w3148]
          tunnel: [w3147] -> w3120 mode=indexing
          tunnel: w3121 -> [w3152] mode=indexing
          tunnel: [w3151] -> w3108 mode=indexing
          tunnel: w3111 -> [w3146]
          n491 = Less?(x=w3154, y=w3157) -> (x < y?=w3156:bool)
          n492 = Index Array(array=w3155, index=w3154) -> (element=w3153:waveform(dbl))
          n493 = case shown="True" w3156 {
            tunnel: w3153 -> [_ w3174]
            tunnel: w3152 -> [w3159 w3172]
            tunnel: [w3159 w3160] -> w3151
            tunnel: w3150 -> [_ w3171]
            tunnel: w3149 -> [_ w3164]
            tunnel: w3148 -> [_ w3163]
            tunnel: [cluster{"f0":dbl, "df":dbl, "magnitude":dbl[]} {"f0"=0.0, "df"=0.0, "magnitude"=[]} ("PSD") w3165] -> w3147
            tunnel: w3146 -> [_ w3162]
            frame #0 {
            }
            frame #1 {
              n494 = call <vilib>:"Std Deviation and Variance.vi"("X"=w3174) -> ("mean"=w3175:dbl)  [unwired: 1 in, 2 out]
              n495 = Subtract(x=w3174, y=w3175) -> (x-y=w3173:waveform(dbl))
              n496 = xnode "Spectral Measurements"("Signals"=w3173) -> ("PSD"=w3167:cluster{"f0":dbl, "df":dbl, "magnitude":dbl[]})  [unwired: 1 in, 1 out]
              n497 = case shown="False" w3171 {
                tunnel: w3172 -> [w3184 _]
                tunnel: [w3180 w3189] -> w3160
                tunnel: w3167 -> [w3183 w3190]
                tunnel: w3164 -> [w3182 _]
                frame #0 {
                  n498 = Build Array (concatenate)(w3184, w3183) -> (w3181:cluster{"f0":dbl, "df":dbl, "magnitude":dbl[]}[])
                  n499 = case shown="True" w3182 {
                    tunnel: w3181 -> [w3185 w3188]
                    tunnel: [w3185 w3186] -> w3180
                    frame #0 {
                    }
                    frame #1 {
                      n500 = Delete From Array(array=w3188, index=0) -> (array with subset deleted=w3186:cluster{"f0":dbl, "df":dbl, "magnitude":dbl[]}[])  [unwired: 1 in, 1 out]
                    }
                  }
                }
                frame #1 {
                  n501 = Build Array(w3190) -> (w3189:cluster{"f0":dbl, "df":dbl, "magnitude":dbl[]}[])
                }
              }
              n502 = for {
                tunnel: w3160 -> [w3179] mode=indexing
                tunnel: [w3178] -> w3170 mode=indexing
                workers-P: _ -> [_]
                n503 = Unbundle By Name(w3179) -> ("magnitude"=w3178:dbl[])
              }
              n504 = Transpose 2D Array(2D array=w3170) -> (transposed array=w3169:dbl[][])
              n505 = for {
                tunnel: w3169 -> [w3177] mode=indexing
                tunnel: [w3176] -> w3168 mode=indexing
                workers-P: _ -> [_]
                n506 = Add Array Elements(numeric array=w3177) -> (sum=w3176:dbl)
              }
              n507 = Select(t=w3163, s=w3164, f=w3162) -> (s? t:f=w3161:dbl)
              n508 = Divide(x=w3168, y=w3161) -> (x/y=w3166:dbl[])
              n509 = Bundle By Name(cluster=w3167, "magnitude"=w3166) -> (w3165:cluster{"f0":dbl, "df":dbl, "magnitude":dbl[]})
            }
          }
        }
        n510 = case shown="True" w3107 {
          tunnel: w3108 -> [w3139 w3145]
          tunnel: [w3139 w3140] -> w3106
          frame #0 {
          }
          frame #1 {
            n511 = Array Subset(array=w3145, index (row)=0 ("index"), length (row)=4 ("length"), index (col)=0 ("index"), length (col)=1 ("length")) -> (w3140:T38)
          }
        }
        n512 = Split 1D Array(array=w3120, index=2) -> (first subarray=→"FFT 1":cluster{"f0":dbl, "df":dbl, "magnitude":dbl[]}[], second subarray=→"FFT 2":cluster{"f0":dbl, "df":dbl, "magnitude":dbl[]}[])
      }
    }
    n513 = Index Array(array=w772, index=1) -> (element=w780:waveform(dbl))
    n514 = case "For displaying the high resolution display (no downsampling)" shown="True" w848 {
      tunnel: w799 -> [_ w1170]
      frame #0 {
      }
      frame #1 {
        n515 = Index Array(array=w1170, index="High Res. Display") -> (element=w1171:waveform(dbl))
        n516 = call <vilib>:"Std Deviation and Variance.vi"("X"=w1171) -> ("mean"=w1178:dbl, "standard deviation"=w1183:dbl)  [unwired: 1 in, 1 out]
        "Mean Intensity" <- w1178
        "Sigma" <- w1183
        n517 = Subtract(x=w1171, y=w1178) -> (x-y=w1177:waveform(dbl))
        n518 = Select(t=w1177, s="Subtract mean", f=w1171) -> (s? t:f=→"1 Channel":waveform(dbl))
        n519 = Divide(x=w1183, y=w1178) -> (x/y=→"Sigma/Mean":dbl)
        n520 = feedback #9(1) -> (w1172:i32)
        n521 = Greater Or Equal?(x=w1172, y="Slow mean N ave.") -> (x >= y?=w1185:bool)
        n522 = Increment(x=w1172) -> (x+1=w1187:i32)
        n523 = Select(t=1, s=w1185, f=w1187) -> (s? t:f=w1174:i32)
        n524 = feedback #10() -> (w1175:waveform(dbl))  [unwired: 1 out]
        n525 = case shown="Default" w1172 {
          tunnel: [w1190 w1193] -> w1176
          tunnel: w1175 -> [w1192 _]
          tunnel: w1171 -> [w1191 w1193]
          frame #0 {
            n526 = call-poly <vilib>:"Append Waveforms.vi"("waveform B"=w1191, "waveform A"=w1192) -> ("waveform out"=w1190:waveform(dbl))  [unwired: 1 in, 8 out]
          }
          frame #1 {
          }
        }
        n527 = case shown="True" w1185 {
          tunnel: w1176 -> [_ w1189]
          frame #0 {
          }
          frame #1 {
            n528 = call <vilib>:"Mean.vi"("X"=w1189) -> ("mean"=→"Slow mean":dbl)  [unwired: 1 out]
          }
        }
      }
    }
    n529 = case "For plotting results of scanning MCL" shown="True" w928 {
      tunnel: w927 -> [_ w1633]
      tunnel: w839 -> [_ w1729]
      tunnel: w936 -> [_ _]
      tunnel: w799 -> [_ w1703]
      tunnel: w774 -> [_ w1634]
      tunnel: w773 -> [_ w1607]
      frame #0 {
      }
      frame #1 {
        w1614 = u32 0 items=["Horizontal", "Vertical", "Central", "1st Diagonal", "2nd Diagonal"] ("Type of Symmetry")
        w1642 = u32 0 items=["Horizontal", "Vertical", "Central", "1st Diagonal", "2nd Diagonal"] ("Type of Symmetry")
        w1645 = u32 0 items=["Horizontal", "Vertical", "Central", "1st Diagonal", "2nd Diagonal"] ("Type of Symmetry")
        w1674 = u32 0 items=["Horizontal", "Vertical", "Central", "1st Diagonal", "2nd Diagonal"] ("Type of Symmetry")
        n530 = Index Array(array=w1703, index=10) -> (element=w1709:waveform(dbl))
        n531 = Index Array(array=w1703, index=11) -> (element=w1706:waveform(dbl))
        n532 = Index Array(array=w1703, index="Channel") -> (element=w1705:waveform(dbl))
        n533 = local read "Cycles/step (MCL)"() -> (w1659:u64)
        n534 = Unbundle(w1607) -> ("New Image"=w1606:T2, "New Image"=w1605:T2, "New Image"=w1604:T2, "New Image"=w1603:T2)
        n535 = Unbundle By Name(w1709) -> ("Y"=w1661:dbl[])
        n536 = Unbundle By Name(w1706) -> ("Y"=w1663:dbl[])
        n537 = Unbundle By Name(w1705) -> ("Y"=w1668:dbl[])
        n538 = call "downsample 1D array - double.vi"("Ave N"=w1659, "Array In"=w1661) -> ("Array Out"=w1660:dbl[])  [unwired: 1 out]
        n539 = call "downsample 1D array - double.vi"("Ave N"=w1659, "Array In"=w1663) -> ("Array Out"=w1662:dbl[])  [unwired: 1 out]
        n540 = call "downsample 1D array - double.vi"("Ave N"=w1659, "Array In"=w1668) -> ("Array Out"=w1667:dbl[])  [unwired: 1 out]
        n541 = feedback #11(w1729) -> (w1730:dbl[])
        n542 = Build Array (concatenate)(w1730, w1729) -> (w1711:dbl[])
        n543 = feedback #12(w1634) -> (w1636:dbl[])
        n544 = Build Array (concatenate)(w1636, w1634) -> (w1635:dbl[])
        n545 = Select(t=w1729, s=w1633, f=w1711) -> (s? t:f=w1715:dbl[])
        n546 = local read "Scan steps (MCL)"() -> (w1616:u64)
        n547 = Select(t=w1634, s=w1633, f=w1635) -> (s? t:f=w1617:dbl[])
        n548 = local read "Scan lines (y)"() -> (w1602:u64)
        n549 = local read "N APD Samp/step"() -> (w1618:dbl)
        n550 = feedback #13(w1660) -> (w1717:dbl[])
        n551 = Build Array (concatenate)(w1717, w1660) -> (w1708:dbl[])
        n552 = feedback #14(w1667) -> (w1727:dbl[])
        n553 = Build Array (concatenate)(w1727, w1667) -> (w1726:dbl[])
        n554 = feedback #15(w1662) -> (w1719:dbl[])
        n555 = Build Array (concatenate)(w1719, w1662) -> (w1720:dbl[])
        n556 = Select(t=w1660, s=w1633, f=w1708) -> (s? t:f=w1664:dbl[])
        n557 = Select(t=w1667, s=w1633, f=w1726) -> (s? t:f=w1666:dbl[])
        n558 = Select(t=w1662, s=w1633, f=w1720) -> (s? t:f=w1665:dbl[])
        n559 = Multiply(x=w1616, y=u64 2) -> (x*y=w1601:u64)
        n560 = call "integrate 1D array interval - double.vi"("Ave N"=w1618, "Array In"=w1617) -> ("Array Out"=w1629:dbl[])  [unwired: 1 out]
        n561 = call "integrate 1D array interval - double.vi"("Ave N"=w1618, "Array In"=w1715) -> ("Array Out"=w1714:dbl[])  [unwired: 1 out]
        n562 = Array Size(array=w1629) -> (size(s)=w1630:i32)
        n563 = Array Size(array=w1714) -> (size(s)=w1716:i32)
        n564 = Multiply(x=w1602, y=w1601) -> (x*y=w1632:u64)
        n565 = Multiply(x=w1602, y=w1601) -> (x*y=w1724:u64)
        n566 = call <vilib>:"Mean.vi"("X"=w1664) -> ("mean"=w1648:dbl)  [unwired: 1 out]
        n567 = Subtract(x=w1632, y=w1630) -> (x-y=w1623:u64)
        n568 = call <vilib>:"Mean.vi"("X"=w1666) -> ("mean"=w1653:dbl)  [unwired: 1 out]
        n569 = call <vilib>:"Mean.vi"("X"=w1665) -> ("mean"=w1651:dbl)  [unwired: 1 out]
        n570 = call <vilib>:"Mean.vi"("X"=w1629) -> ("mean"=w1620:dbl)  [unwired: 1 out]
        n571 = Subtract(x=w1724, y=w1716) -> (x-y=w1658:u64)
        n572 = call <vilib>:"Mean.vi"("X"=w1714) -> ("mean"=w1655:dbl)  [unwired: 1 out]
        n573 = Initialize Array(1.0 ("element"), w1623) -> (w1619:dbl[])
        n574 = Initialize Array(1.0 ("element"), w1658) -> (w1649:dbl[])
        n575 = Multiply(x=w1619, y=w1620) -> (x*y=w1621:dbl[])
        n576 = Multiply(x=w1649, y=w1651) -> (x*y=w1652:dbl[])
        n577 = Multiply(x=w1649, y=w1653) -> (x*y=w1654:dbl[])
        n578 = Multiply(x=w1649, y=w1648) -> (x*y=w1650:dbl[])
        n579 = Multiply(x=w1649, y=w1655) -> (x*y=w1656:dbl[])
        n580 = Build Array (concatenate)(w1664, w1650) -> (w1718:dbl[])
        n581 = Build Array (concatenate)(w1666, w1654) -> (w1722:dbl[])
        n582 = Build Array (concatenate)(w1665, w1652) -> (w1721:dbl[])
        n583 = Build Array (concatenate)(w1629, w1621) -> (w1631:dbl[])
        n584 = Build Array (concatenate)(w1714, w1656) -> (w1723:dbl[])
        n585 = Reshape Array(w1718, w1602, w1601) -> (w1684:dbl[][])
        n586 = Reshape Array(w1631, w1602, w1601) -> (w1627:dbl[][])
        n587 = Reshape Array(w1722, w1602, w1601) -> (w1676:dbl[][])
        n588 = Reshape Array(w1721, w1602, w1601) -> (w1691:dbl[][])
        n589 = Reshape Array(w1723, w1602, w1601) -> (w1701:dbl[][])
        n590 = Array Subset(array=w1691, index (col)=0 ("index"), length (col)=w1616) -> (w1696:dbl[][])  [unwired: 2 in]
        n591 = Array Subset(array=w1691, index (col)=w1616) -> (w1694:dbl[][])  [unwired: 3 in]
        n592 = Array Subset(array=w1676, index (col)=0 ("index"), length (col)=w1616) -> (w1682:dbl[][])  [unwired: 2 in]
        n593 = Array Subset(array=w1676, index (col)=w1616) -> (w1680:dbl[][])  [unwired: 3 in]
        n594 = Array Subset(array=w1627, index (col)=0 ("index"), length (col)=w1616) -> (w1626:dbl[][])  [unwired: 2 in]
        n595 = Array Subset(array=w1627, index (col)=w1616) -> (w1624:dbl[][])  [unwired: 3 in]
        n596 = Array Subset(array=w1701, index (col)=0 ("index"), length (col)=w1616) -> (w1700:dbl[][])  [unwired: 2 in]
        n597 = Array Subset(array=w1701, index (col)=w1616) -> (w1698:dbl[][])  [unwired: 3 in]
        n598 = Array Subset(array=w1684, index (col)=0 ("index"), length (col)=w1616) -> (w1689:dbl[][])  [unwired: 2 in]
        n599 = Array Subset(array=w1684, index (col)=w1616) -> (w1687:dbl[][])  [unwired: 3 in]
        n600 = for {
          tunnel: w1696 -> [w1738] mode=indexing
          tunnel: [w1737] -> w1695 mode=indexing
          workers-P: _ -> [_]
          n601 = Reverse 1D Array(array=w1738) -> (reversed array=w1737:dbl[])
        }
        n602 = for {
          tunnel: w1682 -> [w1734] mode=indexing
          tunnel: [w1733] -> w1681 mode=indexing
          workers-P: _ -> [_]
          n603 = Reverse 1D Array(array=w1734) -> (reversed array=w1733:dbl[])
        }
        n604 = for {
          tunnel: w1626 -> [w1732] mode=indexing
          tunnel: [w1731] -> w1625 mode=indexing
          workers-P: _ -> [_]
          n605 = Reverse 1D Array(array=w1732) -> (reversed array=w1731:dbl[])
        }
        n606 = for {
          tunnel: w1700 -> [w1740] mode=indexing
          tunnel: [w1739] -> w1699 mode=indexing
          workers-P: _ -> [_]
          n607 = Reverse 1D Array(array=w1740) -> (reversed array=w1739:dbl[])
        }
        n608 = for {
          tunnel: w1689 -> [w1736] mode=indexing
          tunnel: [w1735] -> w1688 mode=indexing
          workers-P: _ -> [_]
          n609 = Reverse 1D Array(array=w1736) -> (reversed array=w1735:dbl[])
        }
        n610 = Index Array(array=w1701, index (row)=0) -> (element=→"Waveform Graph":dbl[])  [unwired: 1 in]
        n611 = Add(x=w1695, y=w1694) -> (x+y=w1693:dbl[][])
        n612 = Add(x=w1681, y=w1680) -> (x+y=w1679:dbl[][])
        n613 = Add(x=w1625, y=w1624) -> (x+y=w1609:dbl[][])
        n614 = Add(x=w1699, y=w1698) -> (x+y=w1673:dbl[][])
        n615 = Add(x=w1688, y=w1687) -> (x+y=w1686:dbl[][])
        n616 = Divide(x=w1679, y=2) -> (x/y=w1677:dbl[][])
        n617 = Divide(x=w1693, y=2) -> (x/y=w1638:dbl[][])
        n618 = Divide(x=w1686, y=2) -> (x/y=w1640:dbl[][])
        n619 = To Single Precision Float(number=w1673) -> (single precision float=w1672:sgl[][])
        n620 = Transpose 2D Array(2D array=w1677) -> (transposed array=→"Data map":dbl[][])
        n621 = To Single Precision Float(number=w1609) -> (single precision float=w1613:sgl[][])